vi "CORDLESS_CAMERA_SETUP.vi"(7 "error in":errorcluster) -> (27 "error out":errorcluster={"status"=TRUE, "code"=-1074360311, "source"="IMAQdx Open Camera.vi"})   [LabVIEW 2014]
uses:
  <vilib>/userdefined/High Color/IMAQdx.ctl
  <vilib>/vision/driver/NI_Vision_Acquisition_Software.lvlib
panel:
  in  "stop":bool
  in  "Session In":T1="cam1"
  out "Image Out":T2(plugin-control)
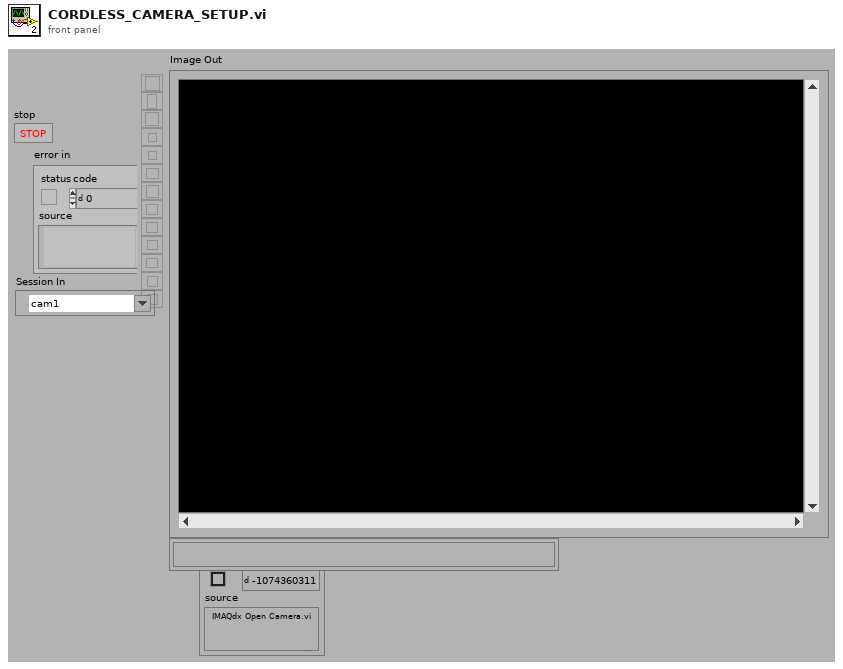
[diagram p1: front panel]
types:
  T1 = typedef "IMAQdx.ctl" = refnum<k21>
  T2 = typedef "IMAQ Image.ctl" = refnum<image>
  T3 = cluster{"Name":string, "Type":enum16{"Line", "Broken Line", "Free Hand Line", "Rotated Rectangle", "Oval", "Polygon", "Free Hand", "Bitmap", "Text"}, "Coordinates":i32[], "Colors":u32[], "Drawing Mode":u32, "Text":string, "Results":cluster{"Process ID":string, "Measure":u16, "Name":string, "String Format":u16, "Width":i16, "Precision":i16, "True String":string, "False String":string}[], "Font, Size & Style":cluster{"Desired Font (Application)":enum16{"User-specified Font", "Application Font", "System Font", "Dialog Font"}, "[User-specified Font]":cluster{"Font Name":string, "Size":i16, "Strikeout?":bool, "Italic?":bool, "Underline?":bool, "Outline?":bool, "Shadow?":bool, "Bold?":bool, "Rotation Angle":dbl}, "Horizontal Alignment":i16, "Vertical Alignment":i16}, "Image File Path":path, "Use Keying Color":bool}[]
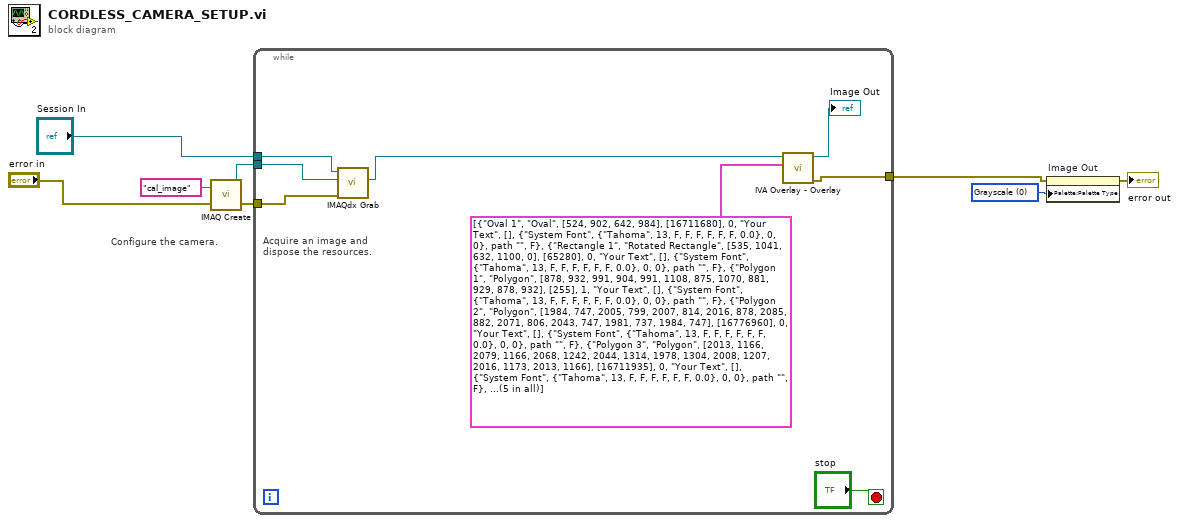
[diagram p0: block diagram]
diagram:
  w6 = u32 0 items=["Grayscale", "Binary", "Gradient", "Rainbow", "Temperature", "User Defined"] ("Palette")
  # "Configure the camera."
  n1 = call "IMAQ Create"("Image Name"="cal_image", "error in (no error)"="error in") -> ("New Image"=w8:T2, "error out"=w7:errorcluster)  [unwired: 2 in, 1 out]
  n2 = while {
    tunnel: w8 -> [w11]
    tunnel: w7 -> [w12]
    tunnel: "Session In" -> [w10]
    tunnel: [w14] -> w1
    stop <- "stop" stop-if-true
    # "Acquire an image and\ndispose the resources."
    n3 = call <vilib>:"IMAQdx Grab.vi"("error in"=w12, "Image In"=w11, "Session In"=w10) -> ("Image Out"=w9:T2)  [unwired: 5 in, 3 out]
    n4 = call <vilib>:"IVA Overlay - Overlay.vi"("Parameters"=T3 [{"Name"="Oval 1", "Type"=enum."Oval", "Coordinates"=[524, 902, 642, 984], "Colors"=[16711680], "Drawing Mode"=0, "Text"="Your Text", "Results"=[], "Font, Size & Style"={"Desired Font (Application)"=enum."System Font", "[User-specified Font]"={"Font Name"="Tahoma", "Size"=13, "Strikeout?"=FALSE, "Italic?"=FALSE, "Underline?"=FALSE, "Outline?"=FALSE, "Shadow?"=FALSE, "Bold?"=FALSE, "Rotation Angle"=0.0}, "Horizontal Alignment"=0, "Vertical Alignment"=0}, "Image File Path"=path "", "Use Keying Color"=FALSE}, {"Name"="Rectangle 1", "Type"=enum."Rotated Rectangle", "Coordinates"=[535, 1041, 632, 1100, 0], "Colors"=[65280], "Drawing Mode"=0, "Text"="Your Text", "Results"=[], "Font, Size & Style"={"Desired Font (Application)"=enum."System Font", "[User-specified Font]"={"Font Name"="Tahoma", "Size"=13, "Strikeout?"=FALSE, "Italic?"=FALSE, "Underline?"=FALSE, "Outline?"=FALSE, "Shadow?"=FALSE, "Bold?"=FALSE, "Rotation Angle"=0.0}, "Horizontal Alignment"=0, "Vertical Alignment"=0}, "Image File Path"=path "", "Use Keying Color"=FALSE}, {"Name"="Polygon 1", "Type"=enum."Polygon", "Coordinates"=[878, 932, 991, 904, 991, 1108, 875, 1070, 881, 929, 878, 932], "Colors"=[255], "Drawing Mode"=1, "Text"="Your Text", "Results"=[], "Font, Size & Style"={"Desired Font (Application)"=enum."System Font", "[User-specified Font]"={"Font Name"="Tahoma", "Size"=13, "Strikeout?"=FALSE, "Italic?"=FALSE, "Underline?"=FALSE, "Outline?"=FALSE, "Shadow?"=FALSE, "Bold?"=FALSE, "Rotation Angle"=0.0}, "Horizontal Alignment"=0, "Vertical Alignment"=0}, "Image File Path"=path "", "Use Keying Color"=FALSE}, {"Name"="Polygon 2", "Type"=enum."Polygon", "Coordinates"=[1984, 747, 2005, 799, 2007, 814, 2016, 878, 2085, 882, 2071, 806, 2043, 747, 1981, 737, 1984, 747], "Colors"=[16776960], "Drawing Mode"=0, "Text"="Your Text", "Results"=[], "Font, Size & Style"={"Desired Font (Application)"=enum."System Font", "[User-specified Font]"={"Font Name"="Tahoma", "Size"=13, "Strikeout?"=FALSE, "Italic?"=FALSE, "Underline?"=FALSE, "Outline?"=FALSE, "Shadow?"=FALSE, "Bold?"=FALSE, "Rotation Angle"=0.0}, "Horizontal Alignment"=0, "Vertical Alignment"=0}, "Image File Path"=path "", "Use Keying Color"=FALSE}, {"Name"="Polygon 3", "Type"=enum."Polygon", "Coordinates"=[2013, 1166, 2079, 1166, 2068, 1242, 2044, 1314, 1978, 1304, 2008, 1207, 2016, 1173, 2013, 1166], "Colors"=[16711935], "Drawing Mode"=0, "Text"="Your Text", "Results"=[], "Font, Size & Style"={"Desired Font (Application)"=enum."System Font", "[User-specified Font]"={"Font Name"="Tahoma", "Size"=13, "Strikeout?"=FALSE, "Italic?"=FALSE, "Underline?"=FALSE, "Outline?"=FALSE, "Shadow?"=FALSE, "Bold?"=FALSE, "Rotation Angle"=0.0}, "Horizontal Alignment"=0, "Vertical Alignment"=0}, "Image File Path"=path "", "Use Keying Color"=FALSE}], "Image In"=w9) -> ("error out"=w14:errorcluster, "Image Out"=→"Image Out":T2)  [unwired: 1 in, 7 out]
  }
  n5 = property on="Image Out" class="ImageControl"(error in=w1, "Palette:Palette Type"=w6) -> (error out=→"error out":errorcluster)  [unwired: 1 in, 1 out]
